vi "Dresden R2R Sputter 03.02.2018 IY24.vi"() -> ()   [LabVIEW 2009] (continued)
                    n14663 = local read "Semi"() -> (w21180:bool)
                    n14664 = case shown="False" w21180 {
                      frame #0 {
                        n14665 = local write "Cassette_servo_speed_value"(u16 300 ("Cassette_servo_speed_value")) -> ()
                      }
                      frame #1 {
                      }
                    }
                  }
                  frame #1 {
                    n14666 = local read "Semi"() -> (w21182:bool)
                    n14667 = case shown="False" w21182 {
                      frame #0 {
                        n14668 = Wait (ms)(milliseconds to wait=u32 200) -> ()  [unwired: 1 out]
                      }
                      frame #1 {
                      }
                    }
                  }
                  frame #2 {
                    n14669 = local read "Semi"() -> (w21184:bool)
                    n14670 = case shown="False" w21184 {
                      frame #0 {
                        n14671 = local write "Cassette_servo_speed_auto_set"(TRUE ("Cassette_servo_speed_set")) -> ()
                      }
                      frame #1 {
                      }
                    }
                  }
                  frame #3 {
                    n14672 = local read "Semi"() -> (w21186:bool)
                    n14673 = case shown="False" w21186 {
                      frame #0 {
                        n14674 = Wait (ms)(milliseconds to wait=u32 200) -> ()  [unwired: 1 out]
                      }
                      frame #1 {
                      }
                    }
                  }
                  frame #4 {
                    n14675 = local read "Semi"() -> (w21188:bool)
                    n14676 = case shown="False" w21188 {
                      frame #0 {
                        n14677 = local write "CH1_2trns_10"(TRUE ("CH1_2trns_7")) -> ()
                        n14678 = Wait (ms)(milliseconds to wait=u32 500) -> ()  [unwired: 1 out]
                      }
                      frame #1 {
                      }
                    }
                  }
                }
              }
              frame #1 {
              }
            }
          }
          frame #15 {
            # "Casette Servo Start"
            n14679 = local read "Semi"() -> (w21191:bool)
            n14680 = case shown="False" w21191 {
              frame #0 {
                n14681 = stacked-sequence {
                  frame #0 {
                    n14682 = while {
                      i -> [w21197]
                      stop <- w21192 stop-if-true
                      n14683 = Greater?(x=w21197, y=50) -> (0:w21198:bool)
                      n14684 = local read "Casette_servo_start/stop_di"() -> (w21195:bool)
                      n14685 = case shown="True" w21198 {
                        frame #0 {
                        }
                        frame #1 {
                          n14686 = local write "Semi"(TRUE ("Semi")) -> ()
                          n14687 = local write "Error Message"("Transfer process was cancelled.\nPlease check Casette connections." ("Error Message")) -> ()
                        }
                      }
                      n14688 = case shown="False" w21195 {
                        tunnel: [FALSE ("Casette_servo_left_direction_do") TRUE ("Casette_servo_left_direction_do")] -> w21194
                        frame #0 {
                          n14689 = Wait Until Next ms Multiple(millisecond multiple=u32 200) -> ()  [unwired: 1 out]
                          n14690 = local write "Casette_servo_start/stop_do"(TRUE ("Casette_servo_left_direction_do")) -> ()
                        }
                        frame #1 {
                        }
                      }
                      n14691 = local read "Semi"() -> (w21193:bool)
                      n14692 = Or(x=w21194, y=w21193) -> (x .or. y?=w21192:bool)
                    }
                  }
                  frame #1 {
                    n14693 = local read "Semi"() -> (w21205:bool)
                    n14694 = case shown="False" w21205 {
                      frame #0 {
                        n14695 = local write "CH1_2trns_11"(TRUE ("CH1_2trns_9")) -> ()
                        n14696 = Wait (ms)(milliseconds to wait=u32 500) -> ()  [unwired: 1 out]
                      }
                      frame #1 {
                      }
                    }
                  }
                }
              }
              frame #1 {
              }
            }
          }
          frame #16 {
            # "SET CASSETTE SERVO  SPEED 100"
            n14697 = local read "Semi"() -> (w21208:bool)
            n14698 = case shown="False" w21208 {
              frame #0 {
                n14699 = stacked-sequence {
                  frame #0 {
                    n14700 = while {
                      i -> [w21215]
                      stop <- w21211 stop-if-true
                      n14701 = local read "Ch3_Right_slow_di"() -> (w21209:bool)
                      n14702 = Greater?(x=w21215, y=1500) -> (0:w21214:bool)
                      n14703 = case shown="True" w21214 {
                        frame #0 {
                        }
                        frame #1 {
                          n14704 = local write "Semi"(TRUE ("Semi")) -> ()
                          n14705 = local write "Error Message"("Transfer process was cancelled.\nPlease check Casette & Sensor\nconnections." ("Error Message")) -> ()
                        }
                      }
                      n14706 = case shown="False" w21209 {
                        tunnel: [FALSE TRUE] -> w21212
                        frame #0 {
                          n14707 = Wait Until Next ms Multiple(millisecond multiple=u32 200) -> ()  [unwired: 1 out]
                        }
                        frame #1 {
                        }
                      }
                      n14708 = local read "Semi"() -> (w21210:bool)
                      n14709 = Or(x=w21212, y=w21210) -> (x .or. y?=w21211:bool)
                    }
                  }
                  frame #1 {
                    n14710 = disable-structure shown="Disabled" {
                      frame #0 {
                        n14711 = while {
                          i -> [w21230]
                          stop <- w21226 stop-if-true
                          n14712 = local read "Counter_read_data"() -> (w21223:i16)
                          n14713 = Greater?(x=w21230, y=5000) -> (0:w21229:bool)
                          n14714 = case shown="True" w21229 {
                            frame #0 {
                            }
                            frame #1 {
                              n14715 = local write "Semi"(TRUE ("Semi")) -> ()
                            }
                          }
                          n14716 = In Range and Coerce(upper limit=i16 1990, x=w21223, lower limit=i16 1980 ("upper limit")) -> (In Range?=w21221:bool)  [unwired: 1 out]
                          n14717 = case shown="True" w21221 {
                            tunnel: [FALSE TRUE] -> w21227
                            frame #0 {
                              n14718 = Wait Until Next ms Multiple(millisecond multiple=u32 200) -> ()  [unwired: 1 out]
                            }
                            frame #1 {
                            }
                          }
                          n14719 = local read "Semi"() -> (w21225:bool)
                          n14720 = Or(x=w21227, y=w21225) -> (x .or. y?=w21226:bool)
                        }
                      }
                      frame #1 {
                      }
                    }
                  }
                  frame #2 {
                    n14721 = local read "Semi"() -> (w21235:bool)
                    n14722 = case shown="False" w21235 {
                      frame #0 {
                        n14723 = local write "Cassette_servo_speed_value"(u16 100 ("Cassette_servo_speed_value")) -> ()
                      }
                      frame #1 {
                      }
                    }
                  }
                  frame #3 {
                    n14724 = local read "Semi"() -> (w21237:bool)
                    n14725 = case shown="False" w21237 {
                      frame #0 {
                        n14726 = Wait (ms)(milliseconds to wait=u32 200 ("millisecond multiple")) -> ()  [unwired: 1 out]
                      }
                      frame #1 {
                      }
                    }
                  }
                  frame #4 {
                    n14727 = local read "Semi"() -> (w21239:bool)
                    n14728 = case shown="False" w21239 {
                      frame #0 {
                        n14729 = local write "Cassette_servo_speed_auto_set"(TRUE ("Cassette_servo_speed_auto_set")) -> ()
                      }
                      frame #1 {
                      }
                    }
                  }
                  frame #5 {
                    n14730 = local read "Semi"() -> (w21241:bool)
                    n14731 = case shown="False" w21241 {
                      frame #0 {
                        n14732 = Wait (ms)(milliseconds to wait=u32 200 ("millisecond multiple")) -> ()  [unwired: 1 out]
                      }
                      frame #1 {
                      }
                    }
                  }
                  frame #6 {
                    n14733 = while {
                      i -> [w21246]
                      stop <- w21243 stop-if-true
                      n14734 = Greater?(x=w21246, y=50) -> (0:w21247:bool)
                      n14735 = local read "Cnt_Right_slow_di"() -> (w21249:bool)
                      n14736 = case shown="True" w21247 {
                        frame #0 {
                        }
                        frame #1 {
                          n14737 = local write "Semi"(TRUE ("Semi")) -> ()
                          n14738 = local write "Error Message"("\nPlease check connections." ("Error Message")) -> ()
                        }
                      }
                      n14739 = case shown="False" w21249 {
                        tunnel: [FALSE ("Cnt_Left_slow_do") TRUE ("Cnt_Left_slow_do")] -> w21245
                        frame #0 {
                          n14740 = local write "Cnt_Right_slow_do"(TRUE ("Cnt_Left_slow_do")) -> ()
                          n14741 = Wait Until Next ms Multiple(millisecond multiple=u32 200) -> ()  [unwired: 1 out]
                        }
                        frame #1 {
                        }
                      }
                      n14742 = local read "Semi"() -> (w21244:bool)
                      n14743 = Or(x=w21245, y=w21244) -> (x .or. y?=w21243:bool)
                    }
                  }
                  frame #7 {
                    n14744 = local read "Semi"() -> (w21256:bool)
                    n14745 = case shown="False" w21256 {
                      frame #0 {
                        n14746 = local write "CH1_2trns_12"(TRUE ("CH1_2trns_11")) -> ()
                        n14747 = Wait (ms)(milliseconds to wait=u32 500) -> ()  [unwired: 1 out]
                      }
                      frame #1 {
                      }
                    }
                  }
                }
              }
              frame #1 {
              }
            }
          }
          frame #17 {
            # "CASETTE STOP AND FIX"
            n14748 = local read "Semi"() -> (w21259:bool)
            n14749 = case shown="False" w21259 {
              frame #0 {
                n14750 = stacked-sequence {
                  frame #0 {
                    # "Center Casette stop"
                    n14751 = local read "Semi"() -> (w21260:bool)
                    n14752 = case shown="False" w21260 {
                      frame #0 {
                        n14753 = stacked-sequence {
                          frame #0 {
                            n14754 = while {
                              i -> [w21267]
                              stop <- w21262 stop-if-true
                              n14755 = local read "Ch3_Right_limit_di"() -> (w21261:bool)
                              n14756 = Greater?(x=w21267, y=600) -> (0:w21265:bool)
                              n14757 = case shown="True" w21265 {
                                frame #0 {
                                }
                                frame #1 {
                                n14758 = local write "Semi"(TRUE ("Semi")) -> ()
                                n14759 = local write "Error Message"("Transfer process was cancelled.\nPlease check Casette connections." ("Error Message")) -> ()
                                }
                              }
                              n14760 = case shown="False" w21261 {
                                tunnel: [FALSE TRUE] -> w21264
                                frame #0 {
                                n14761 = Wait Until Next ms Multiple(millisecond multiple=u32 200) -> ()  [unwired: 1 out]
                                }
                                frame #1 {
                                }
                              }
                              n14762 = local read "Semi"() -> (w21263:bool)
                              n14763 = Or(x=w21264, y=w21263) -> (x .or. y?=w21262:bool)
                            }
                          }
                          frame #1 {
                            n14764 = disable-structure shown="Disabled" {
                              frame #0 {
                                n14765 = while {
                                i -> [w21282]
                                stop <- w21277 stop-if-true
                                n14766 = local read "Counter_read_data"() -> (w21274:i16)
                                n14767 = Greater?(x=w21282, y=5000) -> (0:w21280:bool)
                                n14768 = case shown="True" w21280 {
                                frame #0 {
                                }
                                frame #1 {
                                n14769 = local write "Semi"(TRUE ("Semi")) -> ()
                                n14770 = local write "Error Message"("Transfer process was cancelled.\nPlease check Casette connections." ("Error Message")) -> ()
                                }
                                }
                                n14771 = In Range and Coerce(upper limit=i16 2209, x=w21274, lower limit=i16 2199 ("upper limit")) -> (In Range?=w21273:bool)  [unwired: 1 out]
                                n14772 = case shown="True" w21273 {
                                tunnel: [FALSE TRUE] -> w21279
                                frame #0 {
                                }
                                frame #1 {
                                n14773 = Wait Until Next ms Multiple(millisecond multiple=u32 500) -> ()  [unwired: 1 out]
                                }
                                }
                                n14774 = local read "Semi"() -> (w21278:bool)
                                n14775 = Or(x=w21279, y=w21278) -> (x .or. y?=w21277:bool)
                                }
                              }
                              frame #1 {
                              }
                            }
                          }
                          frame #2 {
                            n14776 = while {
                              i -> [w21294]
                              stop <- w21289 stop-if-true
                              n14777 = local read "Casette_servo_start/stop_di"() -> (w21288:bool)
                              n14778 = Greater?(x=w21294, y=50) -> (0:w21292:bool)
                              n14779 = case shown="True" w21292 {
                                frame #0 {
                                }
                                frame #1 {
                                n14780 = local write "Semi"(TRUE ("Semi")) -> ()
                                n14781 = local write "Error Message"("Transfer process was cancelled.\nPlease check Casette connections." ("Error Message")) -> ()
                                }
                              }
                              n14782 = case shown="True" w21288 {
                                tunnel: [TRUE FALSE] -> w21291
                                frame #0 {
                                }
                                frame #1 {
                                n14783 = Wait Until Next ms Multiple(millisecond multiple=u32 200) -> ()  [unwired: 1 out]
                                n14784 = local write "Casette_servo_start/stop_do"(FALSE ("Casette_servo_start/stop_di")) -> ()
                                }
                              }
                              n14785 = local read "Semi"() -> (w21290:bool)
                              n14786 = Or(x=w21291, y=w21290) -> (x .or. y?=w21289:bool)
                            }
                          }
                          frame #3 {
                            n14787 = local read "Semi"() -> (w21301:bool)
                            n14788 = case shown="False" w21301 {
                              frame #0 {
                                n14789 = Wait (ms)(milliseconds to wait=u32 200) -> ()  [unwired: 1 out]
                              }
                              frame #1 {
                              }
                            }
                          }
                          frame #4 {
                            n14790 = local read "Semi"() -> (w21303:bool)
                            n14791 = case shown="False" w21303 {
                              frame #0 {
                                n14792 = local write "Cassette_servo_speed_value"(u16 0 ("Cassette_servo_speed_value")) -> ()
                              }
                              frame #1 {
                              }
                            }
                          }
                          frame #5 {
                            n14793 = local read "Semi"() -> (w21305:bool)
                            n14794 = case shown="False" w21305 {
                              frame #0 {
                                n14795 = Wait (ms)(milliseconds to wait=u32 200) -> ()  [unwired: 1 out]
                              }
                              frame #1 {
                              }
                            }
                          }
                          frame #6 {
                            n14796 = local read "Semi"() -> (w21307:bool)
                            n14797 = case shown="False" w21307 {
                              frame #0 {
                                n14798 = local write "Cassette_servo_speed_auto_set"(TRUE ("Cassette_servo_speed_auto_set")) -> ()
                              }
                              frame #1 {
                              }
                            }
                          }
                          frame #7 {
                            n14799 = local read "Semi"() -> (w21309:bool)
                            n14800 = case shown="False" w21309 {
                              frame #0 {
                                n14801 = Wait (ms)(milliseconds to wait=u32 200) -> ()  [unwired: 1 out]
                              }
                              frame #1 {
                              }
                            }
                          }
                          frame #8 {
                            n14802 = local read "Semi"() -> (w21311:bool)
                            n14803 = case shown="False" w21311 {
                              frame #0 {
                                n14804 = local write "CH1_2trns_13"(TRUE ("CH1_2trns_9")) -> ()
                                n14805 = Wait (ms)(milliseconds to wait=u32 500) -> ()  [unwired: 1 out]
                              }
                              frame #1 {
                              }
                            }
                          }
                        }
                      }
                      frame #1 {
                      }
                    }
                  }
                  frame #1 {
                    # "CASETTE FIX DOWN CH2"
                    n14806 = local read "Semi"() -> (w21314:bool)
                    n14807 = case shown="False" w21314 {
                      frame #0 {
                        n14808 = stacked-sequence {
                          frame #0 {
                            n14809 = local read "Semi"() -> (w21315:bool)
                            n14810 = case shown="False" w21315 {
                              frame #0 {
                                n14811 = while {
                                i -> [w21322]
                                stop <- w21317 stop-if-true
                                n14812 = Greater?(x=w21322, y=50) -> (0:w21320:bool)
                                n14813 = local read "Ch3_Cst_fix_down_di"() -> (w21316:bool)
                                n14814 = case shown="True" w21320 {
                                frame #0 {
                                }
                                frame #1 {
                                n14815 = local write "Semi"(TRUE ("Semi")) -> ()
                                n14816 = local write "Error Message"("Up/Down positions could not reach\nthe down position.\nPlease check connections." ("Error Message")) -> ()
                                }
                                }
                                n14817 = case shown="False" w21316 {
                                tunnel: [FALSE TRUE] -> w21319
                                frame #0 {
                                n14818 = Wait Until Next ms Multiple(millisecond multiple=u32 200) -> ()  [unwired: 1 out]
                                n14819 = local write "Ch3_Cst_fix_do"(TRUE ("Ch1_pet_cool_up_do")) -> ()
                                }
                                frame #1 {
                                }
                                }
                                n14820 = local read "Semi"() -> (w21318:bool)
                                n14821 = Or(x=w21319, y=w21318) -> (x .or. y?=w21317:bool)
                                }
                              }
                              frame #1 {
                              }
                            }
                          }
                          frame #1 {
                            n14822 = local read "Semi"() -> (w21329:bool)
                            n14823 = case shown="False" w21329 {
                              frame #0 {
                                n14824 = local write "CH1_2trns_14"(TRUE ("CH1_2trns_9")) -> ()
                                n14825 = Wait (ms)(milliseconds to wait=u32 500) -> ()  [unwired: 1 out]
                              }
                              frame #1 {
                              }
                            }
                          }
                        }
                      }
                      frame #1 {
                      }
                    }
                  }
                  frame #2 {
                    n14826 = local read "Semi"() -> (w21332:bool)
                    n14827 = case shown="False" w21332 {
                      frame #0 {
                        n14828 = stacked-sequence {
                          frame #0 {
                            n14829 = local read "Semi"() -> (w21333:bool)
                            n14830 = case shown="False" w21333 {
                              frame #0 {
                                n14831 = while {
                                i -> [w21340]
                                stop <- w21335 stop-if-true
                                n14832 = Greater?(x=w21340, y=50) -> (0:w21338:bool)
                                n14833 = local read "Ch4_Trns_gv_bp_di"() -> (w21334:bool)
                                n14834 = case shown="True" w21338 {
                                frame #0 {
                                }
                                frame #1 {
                                n14835 = local write "Semi"(TRUE ("Semi")) -> ()
                                n14836 = local write "Error Message"("Transfer process was cancelled.\nPlease check CH1-Trns-GV connections." ("Error Message")) -> ()
                                }
                                }
                                n14837 = case shown="True" w21334 {
                                tunnel: [TRUE FALSE] -> w21337
                                frame #0 {
                                }
                                frame #1 {
                                n14838 = Wait Until Next ms Multiple(millisecond multiple=u32 200) -> ()  [unwired: 1 out]
                                n14839 = local write "Ch4_Trns_gv_bp_do"(FALSE ("Ch1_pet_cool_up_do")) -> ()
                                }
                                }
                                n14840 = local read "Semi"() -> (w21336:bool)
                                n14841 = Or(x=w21337, y=w21336) -> (x .or. y?=w21335:bool)
                                }
                              }
                              frame #1 {
                              }
                            }
                          }
                          frame #1 {
                            n14842 = local read "Semi"() -> (w21347:bool)
                            n14843 = case shown="False" w21347 {
                              frame #0 {
                                n14844 = Wait (ms)(milliseconds to wait=u32 500) -> ()  [unwired: 1 out]
                              }
                              frame #1 {
                              }
                            }
                          }
                          frame #2 {
                            n14845 = local read "Semi"() -> (w21349:bool)
                            n14846 = case shown="False" w21349 {
                              frame #0 {
                                n14847 = while {
                                i -> [w21356]
                                stop <- w21351 stop-if-true
                                n14848 = Greater?(x=w21356, y=50) -> (0:w21354:bool)
                                n14849 = local read "Ch3_Trns_gv_bp2_di"() -> (w21350:bool)
                                n14850 = case shown="True" w21354 {
                                frame #0 {
                                }
                                frame #1 {
                                n14851 = local write "Semi"(TRUE ("Semi")) -> ()
                                n14852 = local write "Error Message"("Transfer process was cancelled.\nPlease check CH1-Trns-GV connections." ("Error Message")) -> ()
                                }
                                }
                                n14853 = case shown="True" w21350 {
                                tunnel: [TRUE FALSE] -> w21353
                                frame #0 {
                                }
                                frame #1 {
                                n14854 = local write "Ch3_Trns_gv_bp2_do"(FALSE ("Ch1_pet_cool_up_do")) -> ()
                                n14855 = Wait Until Next ms Multiple(millisecond multiple=u32 200) -> ()  [unwired: 1 out]
                                }
                                }
                                n14856 = local read "Semi"() -> (w21352:bool)
                                n14857 = Or(x=w21353, y=w21352) -> (x .or. y?=w21351:bool)
                                }
                              }
                              frame #1 {
                              }
                            }
                          }
                          frame #3 {
                            n14858 = local read "Semi"() -> (w21363:bool)
                            n14859 = case shown="False" w21363 {
                              frame #0 {
                                n14860 = Wait (ms)(milliseconds to wait=u32 500) -> ()  [unwired: 1 out]
                              }
                              frame #1 {
                              }
                            }
                          }
                        }
                      }
                      frame #1 {
                      }
                    }
                  }
                  frame #3 {
                    n14861 = local read "Semi"() -> (w21365:bool)
                    n14862 = case shown="False" w21365 {
                      frame #0 {
                        n14863 = stacked-sequence {
                          frame #0 {
                            n14864 = local read "Semi"() -> (w21366:bool)
                            n14865 = case shown="False" w21366 {
                              frame #0 {
                                n14866 = local write "Ch3_Trns_gv_open_do"(FALSE ("Ch1_pet_cool_up_do")) -> ()
                              }
                              frame #1 {
                              }
                            }
                          }
                          frame #1 {
                            n14867 = local read "Semi"() -> (w21368:bool)
                            n14868 = case shown="False" w21368 {
                              frame #0 {
                                n14869 = while {
                                i -> [w21375]
                                stop <- w21370 stop-if-true
                                n14870 = Greater?(x=w21375, y=500) -> (0:w21373:bool)
                                n14871 = local read "Ch3_Trns_gv_close_di"() -> (w21369:bool)
                                n14872 = case shown="True" w21373 {
                                frame #0 {
                                }
                                frame #1 {
                                n14873 = local write "Semi"(TRUE ("Semi")) -> ()
                                n14874 = local write "Error Message"("Transfer process was cancelled.\nPlease check  GV connections." ("Error Message")) -> ()
                                }
                                }
                                n14875 = case shown="False" w21369 {
                                tunnel: [FALSE TRUE] -> w21372
                                frame #0 {
                                n14876 = Wait Until Next ms Multiple(millisecond multiple=u32 200) -> ()  [unwired: 1 out]
                                n14877 = local write "Ch3_Trns_gv_close_do"(TRUE ("Ch1_pet_cool_up_do")) -> ()
                                }
                                frame #1 {
                                }
                                }
                                n14878 = local read "Semi"() -> (w21371:bool)
                                n14879 = Or(x=w21372, y=w21371) -> (x .or. y?=w21370:bool)
                                }
                              }
                              frame #1 {
                              }
                            }
                          }
                          frame #2 {
                            n14880 = local read "Semi"() -> (w21382:bool)
                            n14881 = case shown="False" w21382 {
                              frame #0 {
                                n14882 = local write "CH1_2trns_17"(TRUE ("CH1_2trns_9")) -> ()
                                n14883 = Wait (ms)(milliseconds to wait=u32 500) -> ()  [unwired: 1 out]
                              }
                              frame #1 {
                              }
                            }
                          }
                        }
                      }
                      frame #1 {
                      }
                    }
                  }
                  frame #4 {
                    # "PET COOL DOWN OF CH2"
                    n14884 = local read "Semi"() -> (w21385:bool)
                    n14885 = case shown="False" w21385 {
                      frame #0 {
                        n14886 = stacked-sequence {
                          frame #0 {
                            n14887 = local read "Semi"() -> (w21386:bool)
                            n14888 = case shown="False" w21386 {
                              frame #0 {
                                n14889 = local write "Ch3_Pet_cool_up_do"(FALSE ("Ch1_pet_cool_up_do")) -> ()
                              }
                              frame #1 {
                              }
                            }
                          }
                          frame #1 {
                            n14890 = local read "Semi"() -> (w21388:bool)
                            n14891 = case shown="False" w21388 {
                              frame #0 {
                                n14892 = while {
                                i -> [w21395]
                                stop <- w21390 stop-if-true
                                n14893 = Greater?(x=w21395, y=300) -> (0:w21393:bool)
                                n14894 = case shown="True" w21393 {
                                frame #0 {
                                }
                                frame #1 {
                                n14895 = local write "Semi"(TRUE ("Semi")) -> ()
                                n14896 = local write "Error Message"("SBS Cool Up/Down positions could not reach\nthe down position.\nPlease check connections." ("Error Message")) -> ()
                                }
                                }
                                n14897 = local read "Ch3_Pet_cool_down_di"() -> (w21389:bool)
                                n14898 = case shown="False" w21389 {
                                tunnel: [FALSE TRUE] -> w21392
                                frame #0 {
                                n14899 = Wait Until Next ms Multiple(millisecond multiple=u32 200) -> ()  [unwired: 1 out]
                                n14900 = local write "Ch3_Pet_cool_down_do"(TRUE ("Ch1_pet_cool_up_do")) -> ()
                                }
                                frame #1 {
                                }
                                }
                                n14901 = local read "Semi"() -> (w21391:bool)
                                n14902 = Or(x=w21392, y=w21391) -> (x .or. y?=w21390:bool)
                                }
                              }
                              frame #1 {
                              }
                            }
                          }
                          frame #2 {
                            n14903 = local read "Semi"() -> (w21402:bool)
                            n14904 = case shown="False" w21402 {
                              frame #0 {
                                n14905 = local write "CH1_2trns_15"(TRUE ("CH1_2trns_9")) -> ()
                                n14906 = Wait (ms)(milliseconds to wait=u32 500) -> ()  [unwired: 1 out]
                              }
                              frame #1 {
                              }
                            }
                          }
                        }
                      }
                      frame #1 {
                      }
                    }
                  }
                  frame #5 {
                    # "SRV PIS FOR"
                    n14907 = local read "Semi"() -> (w21405:bool)
                    n14908 = case shown="False" w21405 {
                      frame #0 {
                        n14909 = stacked-sequence {
                          frame #0 {
                            n14910 = local read "Semi"() -> (w21406:bool)
                            n14911 = case shown="False" w21406 {
                              frame #0 {
                                n14912 = local write "Ch3_SRV1_PIST_Back_do"(FALSE ("Ch1_pet_cool_up_do")) -> ()
                              }
                              frame #1 {
                              }
                            }
                          }
                          frame #1 {
                            n14913 = local read "Semi"() -> (w21408:bool)
                            n14914 = case shown="False" w21408 {
                              frame #0 {
                                n14915 = while {
                                i -> [w21415]
                                stop <- w21410 stop-if-true
                                n14916 = Greater?(x=w21415, y=100) -> (0:w21413:bool)
                                n14917 = local read "Ch3_SRV1_PIST For_di"() -> (w21409:bool)
                                n14918 = case shown="True" w21413 {
                                frame #0 {
                                }
                                frame #1 {
                                n14919 = local write "Semi"(TRUE ("Semi")) -> ()
                                n14920 = local write "Error Message"("For/Back positions could not reach\nthe forward position.\nPlease check connections." ("Error Message")) -> ()
                                }
                                }
                                n14921 = case shown="False" w21409 {
                                tunnel: [FALSE TRUE] -> w21412
                                frame #0 {
                                n14922 = Wait Until Next ms Multiple(millisecond multiple=u32 200) -> ()  [unwired: 1 out]
                                n14923 = local write "Ch3_SRV1_PIST For_do"(TRUE ("Ch1_pet_cool_up_do")) -> ()
                                }
                                frame #1 {
                                }
                                }
                                n14924 = local read "Semi"() -> (w21411:bool)
                                n14925 = Or(x=w21412, y=w21411) -> (x .or. y?=w21410:bool)
                                }
                              }
                              frame #1 {
                              }
                            }
                          }
                          frame #2 {
                            n14926 = local read "Semi"() -> (w21422:bool)
                            n14927 = case shown="False" w21422 {
                              frame #0 {
                                n14928 = local write "CH1_2trns_16"(TRUE ("CH1_2trns_9")) -> ()
                                n14929 = Wait (ms)(milliseconds to wait=u32 500) -> ()  [unwired: 1 out]
                              }
                              frame #1 {
                              }
                            }
                          }
                        }
                      }
                      frame #1 {
                      }
                    }
                  }
                }
              }
              frame #1 {
              }
            }
          }
          frame #18 {
            # "Sensors deactive"
            n14930 = local read "Semi"() -> (w21425:bool)
            n14931 = case shown="False" w21425 {
              frame #0 {
                n14932 = stacked-sequence {
                  frame #0 {
                    n14933 = local read "Semi"() -> (w21426:bool)
                    n14934 = case shown="False" w21426 {
                      frame #0 {
                        n14935 = while {
                          i -> [w21429]
                          stop <- w21430 stop-if-true
                          n14936 = Greater?(x=w21429, y=50) -> (0:w21427:bool)
                          n14937 = local read "Cnt_Right_slow_di"() -> (w21433:bool)
                          n14938 = case shown="True" w21427 {
                            frame #0 {
                            }
                            frame #1 {
                              n14939 = local write "Semi"(TRUE ("Semi")) -> ()
                              n14940 = local write "Error Message"("Transfer process was\ncancelled.Please check right slow sensor." ("Error Message")) -> ()
                            }
                          }
                          n14941 = case shown="False" w21433 {
                            tunnel: [FALSE ("Ch1_pet_cool_up_do") TRUE ("Ch1_pet_cool_up_do")] -> w21432
                            frame #0 {
                              n14942 = Wait Until Next ms Multiple(millisecond multiple=u32 200) -> ()  [unwired: 1 out]
                              n14943 = local write "Cnt_Right_slow_do"(TRUE ("Ch1_pet_cool_up_do")) -> ()
                            }
                            frame #1 {
                            }
                          }
                          n14944 = local read "Semi"() -> (w21431:bool)
                          n14945 = Or(x=w21432, y=w21431) -> (x .or. y?=w21430:bool)
                        }
                      }
                      frame #1 {
                      }
                    }
                  }
                  frame #1 {
                    n14946 = local read "Semi"() -> (w21440:bool)
                    n14947 = case shown="False" w21440 {
                      frame #0 {
                        n14948 = while {
                          i -> [w21443]
                          stop <- w21444 stop-if-true
                          n14949 = Greater?(x=w21443, y=50) -> (0:w21441:bool)
                          n14950 = local read "Cnt_Right_limit_di"() -> (w21447:bool)
                          n14951 = case shown="True" w21441 {
                            frame #0 {
                            }
                            frame #1 {
                              n14952 = local write "Semi"(TRUE ("Semi")) -> ()
                              n14953 = local write "Error Message"("Transfer process was\ncancelled.Please check right limit sensor." ("Error Message")) -> ()
                            }
                          }
                          n14954 = case shown="False" w21447 {
                            tunnel: [FALSE ("Ch1_pet_cool_up_do") TRUE ("Ch1_pet_cool_up_do")] -> w21446
                            frame #0 {
                              n14955 = Wait Until Next ms Multiple(millisecond multiple=u32 200) -> ()  [unwired: 1 out]
                              n14956 = local write "Cnt_Right_limit_do"(TRUE ("Ch1_pet_cool_up_do")) -> ()
                            }
                            frame #1 {
                            }
                          }
                          n14957 = local read "Semi"() -> (w21445:bool)
                          n14958 = Or(x=w21446, y=w21445) -> (x .or. y?=w21444:bool)
                        }
                      }
                      frame #1 {
                      }
                    }
                  }
                  frame #2 {
                    n14959 = local read "Semi"() -> (w21454:bool)
                    n14960 = case shown="False" w21454 {
                      frame #0 {
                        n14961 = while {
                          i -> [w21457]
                          stop <- w21458 stop-if-true
                          n14962 = Greater?(x=w21457, y=50) -> (0:w21455:bool)
                          n14963 = local read "Cnt_Left_slow_di"() -> (w21461:bool)
                          n14964 = case shown="True" w21455 {
                            frame #0 {
                            }
                            frame #1 {
                              n14965 = local write "Semi"(TRUE ("Semi")) -> ()
                              n14966 = local write "Error Message"("Transfer process was\ncancelled.Please check left slow sensor." ("Error Message")) -> ()
                            }
                          }
                          n14967 = case shown="False" w21461 {
                            tunnel: [FALSE ("Ch1_pet_cool_up_do") TRUE ("Ch1_pet_cool_up_do")] -> w21460
                            frame #0 {
                              n14968 = Wait Until Next ms Multiple(millisecond multiple=u32 200) -> ()  [unwired: 1 out]
                              n14969 = local write "Cnt_Left_slow_do"(TRUE ("Ch1_pet_cool_up_do")) -> ()
                            }
                            frame #1 {
                            }
                          }
                          n14970 = local read "Semi"() -> (w21459:bool)
                          n14971 = Or(x=w21460, y=w21459) -> (x .or. y?=w21458:bool)
                        }
                      }
                      frame #1 {
                      }
                    }
                  }
                  frame #3 {
                    n14972 = local read "Semi"() -> (w21468:bool)
                    n14973 = case shown="False" w21468 {
                      frame #0 {
                        n14974 = while {
                          i -> [w21471]